vi "FlexMag - 23-03-2023.vi"() -> ()   [LabVIEW 2018] (continued)
        n1562 = local read "CH4_M3_D3_DO"() -> (w2043:bool)
        n1563 = feedback #54() -> (w2099:bool)  [unwired: 1 in]
        n1564 = Exclusive Or(1:w2102, 2:w2101) -> (0:w2098:bool)
        n1565 = feedback #55() -> (w2106:bool)  [unwired: 1 in]
        n1566 = Exclusive Or(1:w2103, 2:w2104) -> (0:w2107:bool)
        n1567 = feedback #56() -> (w2116:bool)  [unwired: 1 in]
        n1568 = Exclusive Or(1:w2113, 2:w2114) -> (0:w2117:bool)
        n1569 = feedback #57() -> (w2109:bool)  [unwired: 1 in]
        n1570 = Exclusive Or(1:w2112, 2:w2111) -> (0:w2108:bool)
        n1571 = feedback #58() -> (w2053:bool)  [unwired: 1 in]
        n1572 = Exclusive Or(1:w2056, 2:w2055) -> (0:w2052:bool)
        n1573 = feedback #59() -> (w2045:bool)  [unwired: 1 in]
        n1574 = Exclusive Or(1:w2042, 2:w2043) -> (0:w2046:bool)
        n1575 = feedback #60() -> (w2048:bool)  [unwired: 1 in]
        n1576 = Exclusive Or(1:w2051, 2:w2050) -> (0:w2047:bool)
        n1577 = case shown="True" w2098 {
          tunnel: w2099 -> [_ w2204]
          tunnel: [TRUE FALSE] -> w2100
          tunnel: [FALSE w2205] -> w2083
          frame False {
          }
          frame True {
            n1578 = call "Elapsed Time134"("Reset"=w2204) -> ("Elapsed Time (s)"=w2206:dbl)  [unwired: 11 in, 7 out]
            n1579 = Greater Or Equal?(x=w2206, y=5.0) -> (x >= y?=w2205:bool)
          }
        }
        n1580 = feedback-in #54(w2100) -> ()
        n1581 = case shown="True" w2107 {
          tunnel: w2106 -> [_ w2197]
          tunnel: [TRUE FALSE] -> w2105
          tunnel: [FALSE w2198] -> w2085
          frame False {
          }
          frame True {
            n1582 = call "Elapsed Time135"("Reset"=w2197) -> ("Elapsed Time (s)"=w2199:dbl)  [unwired: 11 in, 7 out]
            n1583 = Greater Or Equal?(x=w2199, y=5.0) -> (x >= y?=w2198:bool)
          }
        }
        n1584 = feedback-in #55(w2105) -> ()
        n1585 = case shown="True" w2117 {
          tunnel: w2116 -> [_ w2218]
          tunnel: [TRUE FALSE] -> w2115
          tunnel: [FALSE w2219] -> w2087
          frame False {
          }
          frame True {
            n1586 = call "Elapsed Time132"("Reset"=w2218) -> ("Elapsed Time (s)"=w2220:dbl)  [unwired: 11 in, 7 out]
            n1587 = Greater Or Equal?(x=w2220, y=5.0) -> (x >= y?=w2219:bool)
          }
        }
        n1588 = feedback-in #56(w2115) -> ()
        n1589 = case shown="True" w2108 {
          tunnel: w2109 -> [_ w2211]
          tunnel: [TRUE FALSE] -> w2110
          tunnel: [FALSE w2212] -> w2084
          frame False {
          }
          frame True {
            n1590 = call "Elapsed Time133"("Reset"=w2211) -> ("Elapsed Time (s)"=w2213:dbl)  [unwired: 11 in, 7 out]
            n1591 = Greater Or Equal?(x=w2213, y=5.0) -> (x >= y?=w2212:bool)
          }
        }
        n1592 = feedback-in #57(w2110) -> ()
        n1593 = case shown="True" w2052 {
          tunnel: w2053 -> [_ w2141]
          tunnel: [TRUE FALSE] -> w2054
          tunnel: [FALSE w2142] -> _
          frame False {
          }
          frame True {
            n1594 = call "Elapsed Time145"("Reset"=w2141) -> ("Elapsed Time (s)"=w2143:dbl)  [unwired: 11 in, 7 out]
            n1595 = Greater Or Equal?(x=w2143, y=5.0) -> (x >= y?=w2142:bool)
          }
        }
        n1596 = feedback-in #58(w2054) -> ()
        n1597 = case shown="True" w2046 {
          tunnel: w2045 -> [_ w2127]
          tunnel: [TRUE FALSE] -> w2044
          tunnel: [FALSE w2128] -> _
          frame False {
          }
          frame True {
            n1598 = call "Elapsed Time148"("Reset"=w2127) -> ("Elapsed Time (s)"=w2129:dbl)  [unwired: 11 in, 7 out]
            n1599 = Greater Or Equal?(x=w2129, y=5.0) -> (x >= y?=w2128:bool)
          }
        }
        n1600 = feedback-in #59(w2044) -> ()
        n1601 = case shown="True" w2047 {
          tunnel: w2048 -> [_ w2134]
          tunnel: [TRUE FALSE] -> w2049
          tunnel: [FALSE w2135] -> _
          frame False {
          }
          frame True {
            n1602 = call "Elapsed Time147"("Reset"=w2134) -> ("Elapsed Time (s)"=w2136:dbl)  [unwired: 11 in, 7 out]
            n1603 = Greater Or Equal?(x=w2136, y=5.0) -> (x >= y?=w2135:bool)
          }
        }
        n1604 = feedback-in #60(w2049) -> ()
        n1605 = local write "ch4_ch_vbv_fail"(w2085) -> ()
        n1606 = local write "ch4_mp_fail"(w2087) -> ()
        n1607 = local write "ch4_tp_bv_fail"(w2084) -> ()
        n1608 = local write "ch4_bg_bv_fail"(w2083) -> ()
        n1609 = local read "CH4_SRV1_Piston_Back_DO"() -> (w2075:bool)
        n1610 = local read "CH4_SRV1_Piston_Back_DI"() -> (w2076:bool)
        n1611 = local read "CH4_SRV1_Piston_For_DO"() -> (w2058:bool)
        n1612 = local read "CH4_SRV1_Piston_For_DI"() -> (w2057:bool)
        n1613 = local read "CH4_Trns_BP_Right_DO"() -> (w2039:bool)
        n1614 = local read "CH4_Trns_BP_Right_DI"() -> (w2040:bool)
        n1615 = local read "CH4_PetCool_Up_DO"() -> (w2068:bool)
        n1616 = local read "CH4_PetCool_Up_DI"() -> (w2067:bool)
        n1617 = local read "CH4_PetCool_Down_DO"() -> (w2065:bool)
        n1618 = local read "CH4_PetCool_Down_DI"() -> (w2066:bool)
        n1619 = local read "CH4_Cst_Fix_Down_DI"() -> (w2077:bool)
        n1620 = local read "CH4_PL_VBV_DO"() -> (w2091:bool)
        n1621 = local read "CH4_PL_VBV_DI"() -> (w2092:bool)
        n1622 = local read "CH4_SoV_Ar_DO"() -> (w2094:bool)
        n1623 = local read "CH4_SoV_Ar_DI"() -> (w2093:bool)
        n1624 = local read "CH4_Cst_Fix_DO"() -> (w2078:bool)
        n1625 = feedback #61() -> (w2089:bool)  [unwired: 1 in]
        n1626 = Exclusive Or(1:w2092, 2:w2091) -> (0:w2088:bool)
        n1627 = feedback #62() -> (w2096:bool)  [unwired: 1 in]
        n1628 = Exclusive Or(1:w2093, 2:w2094) -> (0:w2097:bool)
        n1629 = feedback #63() -> (w2080:bool)  [unwired: 1 in]
        n1630 = Exclusive Or(1:w2077, 2:w2078) -> (0:w2081:bool)
        n1631 = feedback #64() -> (w2073:bool)  [unwired: 1 in]
        n1632 = Exclusive Or(1:w2076, 2:w2075) -> (0:w2072:bool)
        n1633 = feedback #65() -> (w2060:bool)  [unwired: 1 in]
        n1634 = Exclusive Or(1:w2057, 2:w2058) -> (0:w2061:bool)
        n1635 = feedback #66() -> (w2063:bool)  [unwired: 1 in]
        n1636 = Exclusive Or(1:w2066, 2:w2065) -> (0:w2062:bool)
        n1637 = feedback #67() -> (w2070:bool)  [unwired: 1 in]
        n1638 = Exclusive Or(1:w2067, 2:w2068) -> (0:w2071:bool)
        n1639 = feedback #68() -> (w2037:bool)  [unwired: 1 in]
        n1640 = Exclusive Or(1:w2040, 2:w2039) -> (0:w2036:bool)
        n1641 = case shown="True" w2088 {
          tunnel: w2089 -> [_ w2190]
          tunnel: [TRUE FALSE] -> w2090
          tunnel: [FALSE w2191] -> w2086
          frame False {
          }
          frame True {
            n1642 = call "Elapsed Time136"("Reset"=w2190) -> ("Elapsed Time (s)"=w2192:dbl)  [unwired: 11 in, 7 out]
            n1643 = Greater Or Equal?(x=w2192, y=5.0) -> (x >= y?=w2191:bool)
          }
        }
        n1644 = feedback-in #61(w2090) -> ()
        n1645 = case shown="True" w2097 {
          tunnel: w2096 -> [_ w2183]
          tunnel: [TRUE FALSE] -> w2095
          tunnel: [FALSE w2184] -> w2082
          frame False {
          }
          frame True {
            n1646 = call "Elapsed Time137"("Reset"=w2183) -> ("Elapsed Time (s)"=w2185:dbl)  [unwired: 11 in, 7 out]
            n1647 = Greater Or Equal?(x=w2185, y=5.0) -> (x >= y?=w2184:bool)
          }
        }
        n1648 = feedback-in #62(w2095) -> ()
        n1649 = case shown="True" w2081 {
          tunnel: w2080 -> [_ w2176]
          tunnel: [TRUE FALSE] -> w2079
          tunnel: [FALSE w2177] -> _
          frame False {
          }
          frame True {
            n1650 = call "Elapsed Time140"("Reset"=w2176) -> ("Elapsed Time (s)"=w2178:dbl)  [unwired: 11 in, 7 out]
            n1651 = Greater Or Equal?(x=w2178, y=20.0) -> (x >= y?=w2177:bool)
          }
        }
        n1652 = feedback-in #63(w2079) -> ()
        n1653 = case shown="True" w2072 {
          tunnel: w2073 -> [_ w2169]
          tunnel: [TRUE FALSE] -> w2074
          tunnel: [FALSE w2170] -> _
          frame False {
          }
          frame True {
            n1654 = call "Elapsed Time141"("Reset"=w2169) -> ("Elapsed Time (s)"=w2171:dbl)  [unwired: 11 in, 7 out]
            n1655 = Greater Or Equal?(x=w2171, y=25.0) -> (x >= y?=w2170:bool)
          }
        }
        n1656 = feedback-in #64(w2074) -> ()
        n1657 = case shown="True" w2061 {
          tunnel: w2060 -> [_ w2148]
          tunnel: [TRUE FALSE] -> w2059
          tunnel: [FALSE w2149] -> _
          frame False {
          }
          frame True {
            n1658 = call "Elapsed Time144"("Reset"=w2148) -> ("Elapsed Time (s)"=w2150:dbl)  [unwired: 11 in, 7 out]
            n1659 = Greater Or Equal?(x=w2150, y=25.0) -> (x >= y?=w2149:bool)
          }
        }
        n1660 = feedback-in #65(w2059) -> ()
        n1661 = case shown="True" w2062 {
          tunnel: w2063 -> [_ w2162]
          tunnel: [TRUE FALSE] -> w2064
          tunnel: [FALSE w2163] -> _
          frame False {
          }
          frame True {
            n1662 = call "Elapsed Time142"("Reset"=w2162) -> ("Elapsed Time (s)"=w2164:dbl)  [unwired: 11 in, 7 out]
            n1663 = Greater Or Equal?(x=w2164, y=25.0) -> (x >= y?=w2163:bool)
          }
        }
        n1664 = feedback-in #66(w2064) -> ()
        n1665 = case shown="True" w2071 {
          tunnel: w2070 -> [_ w2155]
          tunnel: [TRUE FALSE] -> w2069
          tunnel: [FALSE w2156] -> _
          frame False {
          }
          frame True {
            n1666 = call "Elapsed Time143"("Reset"=w2155) -> ("Elapsed Time (s)"=w2157:dbl)  [unwired: 11 in, 7 out]
            n1667 = Greater Or Equal?(x=w2157, y=25.0) -> (x >= y?=w2156:bool)
          }
        }
        n1668 = feedback-in #67(w2069) -> ()
        n1669 = case shown="True" w2036 {
          tunnel: w2037 -> [_ w2120]
          tunnel: [TRUE FALSE] -> w2038
          tunnel: [FALSE w2121] -> w2041
          frame False {
          }
          frame True {
            n1670 = call "Elapsed Time149"("Reset"=w2120) -> ("Elapsed Time (s)"=w2122:dbl)  [unwired: 11 in, 7 out]
            n1671 = Greater Or Equal?(x=w2122, y=10.0) -> (x >= y?=w2121:bool)
          }
        }
        n1672 = feedback-in #68(w2038) -> ()
        n1673 = local write "ch4_gv_bp_right_fail"(w2041) -> ()
        n1674 = local write "ch4_pl_vbv_fail"(w2086) -> ()
        n1675 = local write "ch4_sov_fail"(w2082) -> ()
      }
    }
    n1676 = flat-sequence {
      frame #0 {
        n1677 = local read "CH3_Trns_Gv_Open_DI"() -> (w2328:bool)
        n1678 = local read "CH3_Trns_BP_Right_DI"() -> (w2329:bool)
        n1679 = local read "pcgv1 position"() -> (w2389:i32)
        n1680 = local read "CH1_Trns_Gv_Open_DI"() -> (w2367:bool)
        n1681 = local read "CH3_Trns_BP_Left_DI"() -> (w2330:bool)
        n1682 = local read "CH4_Trns_BP_Right_DI"() -> (w2264:bool)
        n1683 = local read "CH1_Trns_BP_Left_DI"() -> (w2351:bool)
        n1684 = local read "CH2_Trns_Gv_Open_DI"() -> (w2352:bool)
        n1685 = local read "Tp1_stop_cmnd"() -> (w2227:bool)
        n1686 = local read "CH2_Trns_BP_Right_DI"() -> (w2350:bool)
        n1687 = local read "Tp3_stop_cmnd"() -> (w2224:bool)
        n1688 = local read "pcgv3 position"() -> (w2324:i32)
        n1689 = local read "Tp2_stop_cmnd"() -> (w2223:bool)
        n1690 = local read "CH2_Trns_BP_Left_DI"() -> (w2349:bool)
        n1691 = local read "CH2_CH_ATM_DI"() -> (w2361:bool)
        n1692 = local read "CH1_CH_ATM_DI"() -> (w2394:bool)
        n1693 = local read "pcgv4 position"() -> (w2268:i32)
        n1694 = local read "pcgv2 position"() -> (w2356:i32)
        n1695 = local read "CH3_SoV_Ar_DI"() -> (w2327:bool)
        n1696 = local read "CH2_CH_VBV_DI"() -> (w2362:bool)
        n1697 = local read "CH2_PL_ATM_DI"() -> (w2360:bool)
        n1698 = local read "CH1_CH_VBV_DI"() -> (w2395:bool)
        n1699 = local read "CH1_PL_ATM_DI"() -> (w2392:bool)
        n1700 = local read "CH2_PL_VBV_DI"() -> (w2365:bool)
        n1701 = local read "CH1_PL_VBV_DI"() -> (w2393:bool)
        n1702 = local read "CH1_SoV_Ar_DI"() -> (w2368:bool)
        n1703 = local read "CH2_BG_BV_DI"() -> (w2363:bool)
        n1704 = local read "CH1_BG_BV_DI"() -> (w2396:bool)
        n1705 = local read "CH2_TP_BV_DI"() -> (w2364:bool)
        n1706 = local read "CH3_CH_ATM_DI"() -> (w2319:bool)
        n1707 = local read "CH4_SoV_Ar_DI"() -> (w2265:bool)
        n1708 = local read "CH1_TP_BV_DI"() -> (w2397:bool)
        n1709 = local read "CH3_CH_VBV_DI"() -> (w2318:bool)
        n1710 = local read "CH3_PL_ATM_DI"() -> (w2320:bool)
        n1711 = local read "CH2_SoV_Ar_DI"() -> (w2353:bool)
        n1712 = local read "CH3_PL_VBV_DI"() -> (w2315:bool)
        n1713 = local read "CH4_CH_ATM_DI"() -> (w2273:bool)
        n1714 = local read "CH3_BG_BV_DI"() -> (w2317:bool)
        n1715 = local read "CH2_MP_DI"() -> (w2366:bool)
        n1716 = local read "CH3_TP_BV_DI"() -> (w2316:bool)
        n1717 = local read "CH1_MP_DI"() -> (w2398:bool)
        n1718 = local read "CH2_CC_DI"() -> (w2359:bool)
        n1719 = local read "CH4_CH_VBV_DI"() -> (w2274:bool)
        n1720 = local read "CH4_PL_ATM_DI"() -> (w2272:bool)
        n1721 = local read "CH4_PL_VBV_DI"() -> (w2277:bool)
        n1722 = local read "CH4_BG_BV_DI"() -> (w2275:bool)
        n1723 = local read "CH4_TP_BV_DI"() -> (w2276:bool)
        n1724 = local read "CH3_MP_DI"() -> (w2314:bool)
        n1725 = local read "CH3_CC_DI"() -> (w2321:bool)
        n1726 = local read "CH4_MP_DI"() -> (w2278:bool)
        n1727 = local read "CH4_CC_DI"() -> (w2271:bool)
        n1728 = case shown="True" w2227 {
          tunnel: [w2417 w2420] -> w2228
          frame False {
            n1729 = local read "Tp1 speed gui"() -> (w2419:i32)
            n1730 = Greater?(x=w2419, y=250) -> (0:w2417:bool)
          }
          frame True {
            n1731 = local read "Tp1 speed gui"() -> (w2421:i32)
            n1732 = Greater?(x=w2421, y=400) -> (0:w2420:bool)
          }
        }
        n1733 = Greater?(x=w2389, y=10) -> (0:w2388:bool)
        n1734 = Greater?(x=w2389, y=90) -> (0:w2387:bool)
        n1735 = case shown="True" w2223 {
          tunnel: [w2399 w2402] -> w2229
          frame False {
            n1736 = local read "Tp2 speed gui"() -> (w2401:i32)
            n1737 = Greater?(x=w2401, y=250) -> (0:w2399:bool)
          }
          frame True {
            n1738 = local read "Tp2 speed gui"() -> (w2404:i32)
            n1739 = Greater?(x=w2404, y=400) -> (0:w2402:bool)
          }
        }
        n1740 = local write "ch3_sov_gui"(w2327) -> ()
        n1741 = local write "ch3_4_trns_gv_gui"(w2328) -> ()
        n1742 = local write "ch3_gv_bp_right_gui"(w2329) -> ()
        n1743 = local write "ch3_gv_bp_left_gui"(w2330) -> ()
        n1744 = Greater?(x=w2324, y=10) -> (0:w2323:bool)
        n1745 = Greater?(x=w2324, y=90) -> (0:w2322:bool)
        n1746 = local write "ch4_sov_gui"(w2265) -> ()
        n1747 = local write "ch4_gv_bp_right_gui"(w2264) -> ()
        n1748 = local write "ch2_mp_gui"(w2366) -> ()
        n1749 = local write "ch2_tp_bv_gui"(w2364) -> ()
        n1750 = local write "ch2_bg_bv_gui"(w2363) -> ()
        n1751 = local write "ch2_ch_vbv_gui"(w2362) -> ()
        n1752 = local write "ch2_ch_atm_gui"(w2361) -> ()
        n1753 = local write "ch2_pl_vbv_gui"(w2365) -> ()
        n1754 = local write "ch2_pl_atm_gui"(w2360) -> ()
        n1755 = local write "ch2_cc_gui"(w2359) -> ()
        n1756 = case shown="True" w2224 {
          tunnel: [w2405 w2408] -> w2230
          frame False {
            n1757 = local read "Tp3 speed gui"() -> (w2407:i32)
            n1758 = Greater?(x=w2407, y=250) -> (0:w2405:bool)
          }
          frame True {
            n1759 = local read "Tp3 speed gui"() -> (w2410:i32)
            n1760 = Greater?(x=w2410, y=400) -> (0:w2408:bool)
          }
        }
        n1761 = local write "ch1_sov_gui"(w2368) -> ()
        n1762 = local write "ch1_2_trns_gv_gui"(w2367) -> ()
        n1763 = local write "ch1_gv_bp_left_gui"(w2351) -> ()
        n1764 = local write "ch1_mp_gui"(w2398) -> ()
        n1765 = local write "ch1_tp_bv_gui"(w2397) -> ()
        n1766 = local write "ch1_bg_bv_gui"(w2396) -> ()
        n1767 = local write "ch1_ch_vbv_gui"(w2395) -> ()
        n1768 = local write "ch1_ch_atm_gui"(w2394) -> ()
        n1769 = local write "ch1_pl_vbv_gui"(w2393) -> ()
        n1770 = local write "ch1_pl_atm_gui"(w2392) -> ()
        n1771 = local write "ch2_sov_gui"(w2353) -> ()
        n1772 = local write "ch2_3_trns_gv_gui"(w2352) -> ()
        n1773 = local write "ch2_gv_bp_right_gui"(w2350) -> ()
        n1774 = local write "ch2_gv_bp_left_gui"(w2349) -> ()
        n1775 = Greater?(x=w2268, y=10) -> (0:w2269:bool)
        n1776 = Greater?(x=w2268, y=90) -> (0:w2270:bool)
        n1777 = Greater?(x=w2356, y=10) -> (0:w2357:bool)
        n1778 = Greater?(x=w2356, y=90) -> (0:w2358:bool)
        n1779 = local write "ch1_pcgv_half_gui"(w2388) -> ()
        n1780 = local write "ch1_pcgv_gui"(w2387) -> ()
        n1781 = local write "ch3_mp_gui"(w2314) -> ()
        n1782 = local write "ch3_tp_bv_gui"(w2316) -> ()
        n1783 = local write "ch3_bg_bv_gui"(w2317) -> ()
        n1784 = local write "ch3_ch_vbv_gui"(w2318) -> ()
        n1785 = local write "ch3_ch_atm_gui"(w2319) -> ()
        n1786 = local write "ch3_pl_vbv_gui"(w2315) -> ()
        n1787 = local write "ch3_pl_atm_gui"(w2320) -> ()
        n1788 = local write "ch3_cc_gui"(w2321) -> ()
        n1789 = local write "ch4_mp_gui"(w2278) -> ()
        n1790 = local write "ch4_tp_bv_gui"(w2276) -> ()
        n1791 = local write "ch4_bg_bv_gui"(w2275) -> ()
        n1792 = local write "ch4_ch_vbv_gui"(w2274) -> ()
        n1793 = local write "ch4_ch_atm_gui"(w2273) -> ()
        n1794 = local write "ch4_pl_vbv_gui"(w2277) -> ()
        n1795 = local write "ch4_pl_atm_gui"(w2272) -> ()
        n1796 = local write "ch4_cc_gui"(w2271) -> ()
        n1797 = local write "ch3_pcgv_half_gui"(w2323) -> ()
        n1798 = local write "ch3_pcgv_gui"(w2322) -> ()
        n1799 = local write "ch4_pcgv_half_gui"(w2269) -> ()
        n1800 = local write "ch4_pcgv_gui"(w2270) -> ()
        n1801 = local write "ch2_pcgv_half_gui"(w2357) -> ()
        n1802 = local write "ch2_pcgv_gui"(w2358) -> ()
        n1803 = local write "ch2_tp_gui"(w2229) -> ()
        n1804 = local write "ch1_tp_gui"(w2228) -> ()
        n1805 = local read "ch3 pl pg ai(V)"() -> (w2309:dbl)
        n1806 = local read "ch4 pl pg ai(V)"() -> (w2282:dbl)
        n1807 = local read "ch1 pl pg ai(V)"() -> (w2382:dbl)
        n1808 = local read "ch2 pl pg ai(V)"() -> (w2335:dbl)
        n1809 = local read "CH2_CC_DI"() -> (w2346:bool)
        n1810 = local write "ch3_tp_gui"(w2230) -> ()
        n1811 = local read "CH1_CC_DI"() -> (w2371:bool)
        n1812 = local read "CH3_CC_DI"() -> (w2298:bool)
        n1813 = local read "CH4_CC_DI"() -> (w2293:bool)
        n1814 = feedback #69() -> (w2311:bool)  [unwired: 1 in]
        n1815 = feedback #70() -> (w2280:bool)  [unwired: 1 in]
        n1816 = feedback #71() -> (w2347:bool)  [unwired: 1 in]
        n1817 = feedback #72() -> (w2370:bool)  [unwired: 1 in]
        n1818 = feedback #73() -> (w2384:bool)  [unwired: 1 in]
        n1819 = feedback #74() -> (w2333:bool)  [unwired: 1 in]
        n1820 = feedback #75() -> (w2297:bool)  [unwired: 1 in]
        n1821 = Less Or Equal?(x=w2309, y=0.5) -> (x <= y?=w2310:bool)
        n1822 = Less Or Equal?(x=w2282, y=0.5) -> (x <= y?=w2281:bool)
        n1823 = Less Or Equal?(x=w2382, y=0.5) -> (x <= y?=w2383:bool)
        n1824 = Less Or Equal?(x=w2335, y=0.5) -> (x <= y?=w2334:bool)
        n1825 = feedback #76() -> (w2294:bool)  [unwired: 1 in]
        n1826 = case shown="True" w2346 {
          tunnel: w2347 -> [_ w2534]
          tunnel: [TRUE w2533] -> w2348
          tunnel: [FALSE w2529] -> w2240
          tunnel: [FALSE w2528] -> w2331
          frame False {
          }
          frame True {
            n1827 = local read "ch2 cc ai(V)"() -> (w2531:dbl)
            n1828 = Less Or Equal?(x=w2531, y=0.5) -> (x <= y?=w2532:bool)
            n1829 = case shown="True" w2532 {
              tunnel: [TRUE FALSE] -> w2533
              tunnel: w2534 -> [_ w2538]
              tunnel: [FALSE w2539] -> w2529
              tunnel: [TRUE FALSE] -> w2528
              frame False {
              }
              frame True {
                n1830 = call "Elapsed Time69"("Reset"=w2538) -> ("Elapsed Time (s)"=w2541:dbl)  [unwired: 11 in, 7 out]
                n1831 = Greater Or Equal?(x=w2541, y=6.0) -> (x >= y?=w2539:bool)
              }
            }
          }
        }
        n1832 = feedback-in #71(w2348) -> ()
        n1833 = case shown="True" w2310 {
          tunnel: [TRUE FALSE] -> w2312
          tunnel: w2311 -> [_ w2519]
          tunnel: [FALSE w2520] -> w2306
          tunnel: [TRUE FALSE] -> w2307
          frame False {
          }
          frame True {
            n1834 = call "Elapsed Time71"("Reset"=w2519) -> ("Elapsed Time (s)"=w2522:dbl)  [unwired: 11 in, 7 out]
            n1835 = Greater Or Equal?(x=w2522, y=5.0) -> (x >= y?=w2520:bool)
          }
        }
        n1836 = feedback-in #69(w2312) -> ()
        n1837 = case shown="True" w2281 {
          tunnel: [TRUE FALSE] -> w2279
          tunnel: w2280 -> [_ w2482]
          tunnel: [FALSE w2483] -> w2285
          tunnel: [TRUE FALSE] -> w2284
          frame False {
          }
          frame True {
            n1838 = call "Elapsed Time74"("Reset"=w2482) -> ("Elapsed Time (s)"=w2485:dbl)  [unwired: 11 in, 7 out]
            n1839 = Greater Or Equal?(x=w2485, y=5.0) -> (x >= y?=w2483:bool)
          }
        }
        n1840 = feedback-in #70(w2279) -> ()
        n1841 = case shown="True" w2371 {
          tunnel: w2370 -> [_ w2571]
          tunnel: [TRUE w2570] -> w2369
          tunnel: [FALSE w2566] -> w2232
          tunnel: [FALSE w2565] -> w2386
          frame False {
          }
          frame True {
            n1842 = local read "ch1 cc ai(V)"() -> (w2568:dbl)
            n1843 = Less Or Equal?(x=w2568, y=0.5) -> (x <= y?=w2569:bool)
            n1844 = case shown="True" w2569 {
              tunnel: [TRUE FALSE] -> w2570
              tunnel: w2571 -> [_ w2575]
              tunnel: [FALSE w2576] -> w2566
              tunnel: [TRUE FALSE] -> w2565
              frame False {
              }
              frame True {
                n1845 = call "Elapsed Time45"("Reset"=w2575) -> ("Elapsed Time (s)"=w2578:dbl)  [unwired: 11 in, 7 out]
                n1846 = Greater Or Equal?(x=w2578, y=6.0) -> (x >= y?=w2576:bool)
              }
            }
          }
        }
        n1847 = feedback-in #72(w2369) -> ()
        n1848 = case shown="True" w2383 {
          tunnel: [TRUE FALSE] -> w2385
          tunnel: w2384 -> [_ w2593]
          tunnel: [FALSE w2594] -> w2379
          tunnel: [TRUE FALSE] -> w2380
          frame False {
          }
          frame True {
            n1849 = call "Elapsed Time46"("Reset"=w2593) -> ("Elapsed Time (s)"=w2596:dbl)  [unwired: 11 in, 7 out]
            n1850 = Greater Or Equal?(x=w2596, y=5.0) -> (x >= y?=w2594:bool)
          }
        }
        n1851 = feedback-in #73(w2385) -> ()
        n1852 = case shown="True" w2298 {
          tunnel: w2297 -> [_ w2497]
          tunnel: [TRUE w2496] -> w2296
          tunnel: [FALSE w2492] -> w2248
          tunnel: [FALSE w2491] -> w2313
          frame False {
          }
          frame True {
            n1853 = local read "ch3 cc ai(V)"() -> (w2494:dbl)
            n1854 = Less Or Equal?(x=w2494, y=0.5) -> (x <= y?=w2495:bool)
            n1855 = case shown="True" w2495 {
              tunnel: [TRUE FALSE] -> w2496
              tunnel: w2497 -> [_ w2501]
              tunnel: [FALSE w2502] -> w2492
              tunnel: [TRUE FALSE] -> w2491
              frame False {
              }
              frame True {
                n1856 = call "Elapsed Time73"("Reset"=w2501) -> ("Elapsed Time (s)"=w2504:dbl)  [unwired: 11 in, 7 out]
                n1857 = Greater Or Equal?(x=w2504, y=6.0) -> (x >= y?=w2502:bool)
              }
            }
          }
        }
        n1858 = feedback-in #75(w2296) -> ()
        n1859 = case shown="True" w2334 {
          tunnel: [TRUE FALSE] -> w2332
          tunnel: w2333 -> [_ w2556]
          tunnel: [FALSE w2557] -> w2338
          tunnel: [TRUE FALSE] -> w2337
          frame False {
          }
          frame True {
            n1860 = call "Elapsed Time67"("Reset"=w2556) -> ("Elapsed Time (s)"=w2559:dbl)  [unwired: 11 in, 7 out]
            n1861 = Greater Or Equal?(x=w2559, y=5.0) -> (x >= y?=w2557:bool)
          }
        }
        n1862 = feedback-in #74(w2332) -> ()
        n1863 = local read "CH2_CC_DO"() -> (w2243:bool)
        n1864 = local read "CH2_CC_DI"() -> (w2244:bool)
        n1865 = local read "CH1_CC_DO"() -> (w2235:bool)
        n1866 = local read "CH1_CC_DI"() -> (w2236:bool)
        n1867 = local read "CH3_CC_DO"() -> (w2253:bool)
        n1868 = local read "CH3_CC_DI"() -> (w2252:bool)
        n1869 = local read "Tp4_stop_cmnd"() -> (w2226:bool)
        n1870 = case shown="True" w2293 {
          tunnel: w2294 -> [_ w2460]
          tunnel: [TRUE w2459] -> w2295
          tunnel: [FALSE w2455] -> w2257
          tunnel: [FALSE w2454] -> w2258
          frame False {
          }
          frame True {
            n1871 = local read "ch4 cc ai(V)"() -> (w2457:dbl)
            n1872 = Less Or Equal?(x=w2457, y=0.5) -> (x <= y?=w2458:bool)
            n1873 = case shown="True" w2458 {
              tunnel: [TRUE FALSE] -> w2459
              tunnel: w2460 -> [_ w2464]
              tunnel: [FALSE w2465] -> w2455
              tunnel: [TRUE FALSE] -> w2454
              frame False {
              }
              frame True {
                n1874 = call "Elapsed Time76"("Reset"=w2464) -> ("Elapsed Time (s)"=w2467:dbl)  [unwired: 11 in, 7 out]
                n1875 = Greater Or Equal?(x=w2467, y=6.0) -> (x >= y?=w2465:bool)
              }
            }
          }
        }
        n1876 = feedback-in #76(w2295) -> ()
        n1877 = local read "CH4_CC_DO"() -> (w2260:bool)
        n1878 = local read "CH4_CC_DI"() -> (w2261:bool)
        n1879 = feedback #77() -> (w2246:bool)  [unwired: 1 in]
        n1880 = Exclusive Or(1:w2244, 2:w2243) -> (0:w2245:bool)
        n1881 = feedback #78() -> (w2238:bool)  [unwired: 1 in]
        n1882 = Exclusive Or(1:w2236, 2:w2235) -> (0:w2237:bool)
        n1883 = feedback #79() -> (w2250:bool)  [unwired: 1 in]
        n1884 = Exclusive Or(1:w2252, 2:w2253) -> (0:w2251:bool)
        n1885 = case shown="True" w2226 {
          tunnel: [w2411 w2414] -> w2225
          frame False {
            n1886 = local read "Tp4 speed gui"() -> (w2413:i32)
            n1887 = Greater?(x=w2413, y=250) -> (0:w2411:bool)
          }
          frame True {
            n1888 = local read "Tp4 speed gui"() -> (w2416:i32)
            n1889 = Greater?(x=w2416, y=400) -> (0:w2414:bool)
          }
        }
        n1890 = feedback #80() -> (w2263:bool)  [unwired: 1 in]
        n1891 = Exclusive Or(1:w2261, 2:w2260) -> (0:w2262:bool)
        n1892 = case shown="True" w2245 {
          tunnel: w2246 -> [_ w2432]
          tunnel: [TRUE FALSE] -> w2242
          tunnel: [FALSE w2433] -> w2241
          frame False {
          }
          frame True {
            n1893 = call "Elapsed Time86"("Reset"=w2432) -> ("Elapsed Time (s)"=w2434:dbl)  [unwired: 11 in, 7 out]
            n1894 = Greater Or Equal?(x=w2434, y=5.0) -> (x >= y?=w2433:bool)
          }
        }
        n1895 = feedback-in #77(w2242) -> ()
        n1896 = case shown="True" w2237 {
          tunnel: w2238 -> [_ w2425]
          tunnel: [TRUE FALSE] -> w2234
          tunnel: [FALSE w2426] -> w2233
          frame False {
          }
          frame True {
            n1897 = call "Elapsed Time87"("Reset"=w2425) -> ("Elapsed Time (s)"=w2427:dbl)  [unwired: 11 in, 7 out]
            n1898 = Greater Or Equal?(x=w2427, y=5.0) -> (x >= y?=w2426:bool)
          }
        }
        n1899 = feedback-in #78(w2234) -> ()
        n1900 = case shown="True" w2251 {
          tunnel: w2250 -> [_ w2439]
          tunnel: [TRUE FALSE] -> w2254
          tunnel: [FALSE w2440] -> w2249
          frame False {
          }
          frame True {
            n1901 = call "Elapsed Time85"("Reset"=w2439) -> ("Elapsed Time (s)"=w2441:dbl)  [unwired: 11 in, 7 out]
            n1902 = Greater Or Equal?(x=w2441, y=5.0) -> (x >= y?=w2440:bool)
          }
        }
        n1903 = feedback-in #79(w2254) -> ()
        n1904 = local write "ch3_pl_pg_fail"(w2306) -> ()
        n1905 = local write "ch3_pl_pg_gui"(w2307) -> ()
        n1906 = local write "ch4_pl_pg_fail"(w2285) -> ()
        n1907 = local write "ch4_pl_pg_gui"(w2284) -> ()
        n1908 = local write "ch1_pl_pg_fail"(w2379) -> ()
        n1909 = local write "ch1_pl_pg_gui"(w2380) -> ()
        n1910 = local write "ch2_pl_pg_fail"(w2338) -> ()
        n1911 = local write "ch2_pl_pg_gui"(w2337) -> ()
        n1912 = case shown="True" w2262 {
          tunnel: w2263 -> [_ w2446]
          tunnel: [TRUE FALSE] -> w2259
          tunnel: [FALSE w2447] -> w2256
          frame False {
          }
          frame True {
            n1913 = call "Elapsed Time66"("Reset"=w2446) -> ("Elapsed Time (s)"=w2448:dbl)  [unwired: 11 in, 7 out]
            n1914 = Greater Or Equal?(x=w2448, y=5.0) -> (x >= y?=w2447:bool)
          }
        }
        n1915 = feedback-in #80(w2259) -> ()
        n1916 = local read "ch3 ch pg ai(V)"() -> (w2302:dbl)
        n1917 = local read "ch4 ch pg ai(V)"() -> (w2289:dbl)
        n1918 = local read "ch2 ch pg ai(V)"() -> (w2342:dbl)
        n1919 = local read "ch1 ch pg ai(V)"() -> (w2375:dbl)
        n1920 = local write "ch4_tp_gui"(w2225) -> ()
        n1921 = local write "ch1_cc_gui"(w2386) -> ()
        n1922 = local write "ch2_cc_gui"(w2331) -> ()
        n1923 = local write "ch3_cc_gui"(w2313) -> ()
        n1924 = feedback #81() -> (w2300:bool)  [unwired: 1 in]
        n1925 = feedback #82() -> (w2291:bool)  [unwired: 1 in]
        n1926 = feedback #83() -> (w2344:bool)  [unwired: 1 in]
        n1927 = feedback #84() -> (w2373:bool)  [unwired: 1 in]
        n1928 = Less Or Equal?(x=w2302, y=0.5) -> (x <= y?=w2301:bool)
        n1929 = Less Or Equal?(x=w2289, y=0.5) -> (x <= y?=w2290:bool)
        n1930 = Less Or Equal?(x=w2342, y=0.5) -> (x <= y?=w2343:bool)
        n1931 = Less Or Equal?(x=w2375, y=0.5) -> (x <= y?=w2374:bool)
        n1932 = local write "ch4_cc_gui"(w2258) -> ()
        n1933 = case shown="True" w2301 {
          tunnel: [TRUE FALSE] -> w2299
          tunnel: w2300 -> [_ w2510]
          tunnel: [FALSE w2511] -> w2305
          tunnel: [TRUE FALSE] -> w2304
          frame False {
          }
          frame True {
            n1934 = call "Elapsed Time72"("Reset"=w2510) -> ("Elapsed Time (s)"=w2513:dbl)  [unwired: 11 in, 7 out]
            n1935 = Greater Or Equal?(x=w2513, y=5.0) -> (x >= y?=w2511:bool)
          }
        }
        n1936 = feedback-in #81(w2299) -> ()
        n1937 = case shown="True" w2290 {
          tunnel: [TRUE FALSE] -> w2292
          tunnel: w2291 -> [_ w2473]
          tunnel: [FALSE w2474] -> w2286
          tunnel: [TRUE FALSE] -> w2287
          frame False {
          }
          frame True {
            n1938 = call "Elapsed Time75"("Reset"=w2473) -> ("Elapsed Time (s)"=w2476:dbl)  [unwired: 11 in, 7 out]
            n1939 = Greater Or Equal?(x=w2476, y=5.0) -> (x >= y?=w2474:bool)
          }
        }
        n1940 = feedback-in #82(w2292) -> ()
        n1941 = case shown="True" w2343 {
          tunnel: [TRUE FALSE] -> w2345
          tunnel: w2344 -> [_ w2547]
          tunnel: [FALSE w2548] -> w2339
          tunnel: [TRUE FALSE] -> w2340
          frame False {
          }
          frame True {
            n1942 = call "Elapsed Time68"("Reset"=w2547) -> ("Elapsed Time (s)"=w2550:dbl)  [unwired: 11 in, 7 out]
            n1943 = Greater Or Equal?(x=w2550, y=5.0) -> (x >= y?=w2548:bool)
          }
        }
        n1944 = feedback-in #83(w2345) -> ()
        n1945 = case shown="True" w2374 {
          tunnel: [TRUE FALSE] -> w2372
          tunnel: w2373 -> [_ w2584]
          tunnel: [FALSE w2585] -> w2378
          tunnel: [TRUE FALSE] -> w2377
          frame False {
          }
          frame True {
            n1946 = call "Elapsed Time47"("Reset"=w2584) -> ("Elapsed Time (s)"=w2587:dbl)  [unwired: 11 in, 7 out]
            n1947 = Greater Or Equal?(x=w2587, y=5.0) -> (x >= y?=w2585:bool)
          }
        }
        n1948 = feedback-in #84(w2372) -> ()
        n1949 = Or(x=w2232, y=w2233) -> (x .or. y?=w2231:bool)
        n1950 = Or(x=w2240, y=w2241) -> (x .or. y?=w2239:bool)
        n1951 = Or(x=w2248, y=w2249) -> (x .or. y?=w2247:bool)
        n1952 = local write "ch1_cc_fail"(w2231) -> ()
        n1953 = local write "ch2_cc_fail"(w2239) -> ()
        n1954 = Or(x=w2257, y=w2256) -> (x .or. y?=w2255:bool)
        n1955 = local write "ch3_cc_fail"(w2247) -> ()
        n1956 = local write "ch4_cc_fail"(w2255) -> ()
        n1957 = local write "ch3_ch_pg_gui"(w2304) -> ()
        n1958 = local write "ch3_ch_pg_fail"(w2305) -> ()
        n1959 = local write "ch4_ch_pg_gui"(w2287) -> ()
        n1960 = local write "ch4_ch_pg_fail"(w2286) -> ()
        n1961 = local write "ch2_ch_pg_gui"(w2340) -> ()
        n1962 = local write "ch2_ch_pg_fail"(w2339) -> ()
        n1963 = local write "ch1_ch_pg_gui"(w2377) -> ()
        n1964 = local write "ch1_ch_pg_fail"(w2378) -> ()
      }
    }
    n1965 = Wait Until Next ms Multiple(millisecond multiple=u32 300) -> ()  [unwired: 1 out]
  }
  n1966 = local write "Tp4_stop_cmnd"(w19) -> ()
  n1967 = local write "Tp3_stop_cmnd"(w19) -> ()
  n1968 = local write "Tp2_stop_cmnd"(w19) -> ()
  n1969 = local write "Tp1_stop_cmnd"(w19) -> ()
  n1970 = while {
    stop <- FALSE stop-if-true
    n1971 = stacked-sequence {
      seq-local: [w2602 _ _ _ _ _ _] -> [_ w3296 _ _ _ _ _]
      seq-local: [_ _ _ _ w4002 _ _] -> [_ _ _ _ _ _ w5167]
      seq-local: [_ w3019 _ _ _ _ _] -> [_ _ _ _ _ _ w5165]
      seq-local: [_ _ _ _ w3970 _ _] -> [_ _ _ _ _ _ w5158]
      frame #0 {
        n1972 = local read "tp vbv on jpeg"() -> (w2609:u32[][])
        n1973 = local read "pl atm on jpeg"() -> (w2615:u32[][])
        n1974 = local read "pl atm fail jpeg"() -> (w2614:u32[][])
        n1975 = local read "pl pg on jpeg"() -> (w2613:u32[][])
        n1976 = local read "tp vbv fail jpeg"() -> (w2608:u32[][])
        n1977 = local read "pl pg fail jpeg"() -> (w2612:u32[][])
        n1978 = local read "pc gv half jpeg"() -> (w2603:u32[][])
        n1979 = local read "pc gv on jpeg"() -> (w2604:u32[][])
        n1980 = local read "pc gv fail jpeg"() -> (w2605:u32[][])
        n1981 = local read "tp start jpeg"() -> (w2607:u32[][])
        n1982 = local read "main screen jpeg"() -> (w2620:u32[][])
        n1983 = local read "mp on jpeg"() -> (w2619:u32[][])
        n1984 = local read "mp fail jpeg"() -> (w2618:u32[][])
        n1985 = local read "tp fail jpeg"() -> (w2606:u32[][])
        n1986 = local read "tp bv fail jpeg"() -> (w2610:u32[][])
        n1987 = local read "pl vbv on jpeg"() -> (w2617:u32[][])
        n1988 = local read "pl vbv fail jpeg"() -> (w2616:u32[][])
        n1989 = local read "tp bv on jpeg"() -> (w2611:u32[][])
        n1990 = Build Array(FALSE, "ch2_mp_gui", "ch2_mp_fail") -> (w2902:bool[])
        n1991 = Build Array(FALSE, "ch3_mp_gui", "ch3_mp_fail") -> (w2891:bool[])
        n1992 = Build Array(FALSE, "ch4_mp_gui", "ch4_mp_fail") -> (w2885:bool[])
        n1993 = Build Array(FALSE, "ch1_pl_vbv_gui", "ch1_pl_vbv_fail") -> (w2872:bool[])
        n1994 = Build Array(FALSE, "ch1_pl_atm_gui", "ch1_pl_atm_fail") -> (w2808:bool[])
        n1995 = Build Array(FALSE, "ch1_pl_pg_gui", "ch1_pl_pg_fail") -> (w2800:bool[])
        n1996 = Build Array(FALSE, "ch3_pl_vbv_gui", "ch3_pl_vbv_fail") -> (w2861:bool[])
        n1997 = Build Array(FALSE, "ch1_tp_gui", "ch1_tp_fail") -> (w2668:bool[])
        n1998 = Build Array(FALSE, "ch1_tp_bv_gui", "ch1_tp_bv_fail") -> (w2740:bool[])
        n1999 = Build Array(FALSE, "ch1_ch_vbv_gui", "ch1_ch_vbv_fail") -> (w2726:bool[])
        n2000 = Build Array(FALSE, "ch4_pl_vbv_gui", "ch4_pl_vbv_fail") -> (w2857:bool[])
        n2001 = Build Array(FALSE, "ch3_pl_atm_gui", "ch3_pl_atm_fail") -> (w2819:bool[])
        n2002 = Build Array(FALSE, "ch3_pl_pg_gui", "ch3_pl_pg_fail") -> (w2789:bool[])
        n2003 = Build Array(FALSE, "ch3_tp_gui", "ch3_tp_fail") -> (w2679:bool[])
        n2004 = Build Array(FALSE, "ch3_tp_bv_gui", "ch3_tp_bv_fail") -> (w2751:bool[])
        n2005 = Build Array(FALSE, "ch3_ch_vbv_gui", "ch3_ch_vbv_fail") -> (w2715:bool[])
        n2006 = Build Array(FALSE, "ch2_pl_vbv_gui", "ch2_pl_vbv_fail") -> (w2868:bool[])
        n2007 = Build Array(FALSE, "ch4_pl_atm_gui", "ch4_pl_atm_fail") -> (w2823:bool[])
        n2008 = Build Array(FALSE, "ch4_pl_pg_gui", "ch4_pl_pg_fail") -> (w2785:bool[])
        n2009 = Build Array(FALSE, "ch1_mp_gui", "ch1_mp_fail") -> (w2910:bool[])
        n2010 = Build Array(FALSE, "ch4_tp_gui", "ch4_tp_fail") -> (w2683:bool[])
        n2011 = Build Array(FALSE, "ch4_tp_bv_gui", "ch4_tp_bv_fail") -> (w2755:bool[])
        n2012 = Build Array(FALSE, "ch4_ch_vbv_gui", "ch4_ch_vbv_fail") -> (w2711:bool[])
        n2013 = Build Array(FALSE, "ch2_pl_atm_gui", "ch2_pl_atm_fail") -> (w2812:bool[])
        n2014 = Build Array(FALSE, "ch2_pl_pg_gui", "ch2_pl_pg_fail") -> (w2796:bool[])
        n2015 = Build Array(FALSE, "ch2_tp_gui", "ch2_tp_fail") -> (w2672:bool[])
        n2016 = Build Array(FALSE, "ch2_tp_bv_gui", "ch2_tp_bv_fail") -> (w2744:bool[])
        n2017 = Build Array(FALSE, "ch2_ch_vbv_gui", "ch2_ch_vbv_fail") -> (w2722:bool[])
        n2018 = Boolean Array To Number(Boolean array=w2902) -> (number=w2901:u32)
        n2019 = Boolean Array To Number(Boolean array=w2891) -> (number=w2892:u32)
        n2020 = Boolean Array To Number(Boolean array=w2885) -> (number=w2884:u32)
        n2021 = Build Array(FALSE, "ch1_pcgv_half_gui", "ch1_pcgv_gui", "ch1_pcgv_fail") -> (w2653:bool[])
        n2022 = Build Array(FALSE, "ch3_pcgv_half_gui", "ch3_pcgv_gui", "ch3_pcgv_fail") -> (w2642:bool[])
        n2023 = Build Array(FALSE, "ch2_pcgv_half_gui", "ch2_pcgv_gui", "ch2_pcgv_fail") -> (w2649:bool[])
        n2024 = Boolean Array To Number(Boolean array=w2872) -> (number=w2871:u32)
        n2025 = Boolean Array To Number(Boolean array=w2808) -> (number=w2809:u32)
        n2026 = Boolean Array To Number(Boolean array=w2800) -> (number=w2799:u32)
        n2027 = Build Array(FALSE, "ch4_pcgv_half_gui", "ch4_pcgv_gui", "ch4_pcgv_fail") -> (w2638:bool[])
        n2028 = Boolean Array To Number(Boolean array=w2861) -> (number=w2860:u32)
        n2029 = Boolean Array To Number(Boolean array=w2668) -> (number=w2669:u32)
        n2030 = Boolean Array To Number(Boolean array=w2740) -> (number=w2741:u32)
        n2031 = Boolean Array To Number(Boolean array=w2726) -> (number=w2725:u32)
        n2032 = Boolean Array To Number(Boolean array=w2857) -> (number=w2858:u32)
        n2033 = Boolean Array To Number(Boolean array=w2819) -> (number=w2820:u32)
        n2034 = Boolean Array To Number(Boolean array=w2789) -> (number=w2788:u32)
        n2035 = Boolean Array To Number(Boolean array=w2679) -> (number=w2680:u32)
        n2036 = Boolean Array To Number(Boolean array=w2751) -> (number=w2752:u32)
        n2037 = Boolean Array To Number(Boolean array=w2715) -> (number=w2714:u32)
        n2038 = Boolean Array To Number(Boolean array=w2868) -> (number=w2869:u32)
        n2039 = Boolean Array To Number(Boolean array=w2823) -> (number=w2822:u32)
        n2040 = Boolean Array To Number(Boolean array=w2785) -> (number=w2786:u32)
        n2041 = Boolean Array To Number(Boolean array=w2910) -> (number=w2911:u32)
        n2042 = Boolean Array To Number(Boolean array=w2683) -> (number=w2682:u32)
        n2043 = Boolean Array To Number(Boolean array=w2755) -> (number=w2754:u32)
        n2044 = Boolean Array To Number(Boolean array=w2711) -> (number=w2712:u32)
        n2045 = Boolean Array To Number(Boolean array=w2812) -> (number=w2811:u32)
        n2046 = Boolean Array To Number(Boolean array=w2796) -> (number=w2797:u32)
        n2047 = Boolean Array To Number(Boolean array=w2672) -> (number=w2671:u32)
        n2048 = Boolean Array To Number(Boolean array=w2744) -> (number=w2743:u32)
        n2049 = Boolean Array To Number(Boolean array=w2722) -> (number=w2723:u32)
        n2050 = Mantissa & Exponent(0:w2901) -> (2:w2897:dbl)  [unwired: 1 out]
        n2051 = Mantissa & Exponent(0:w2892) -> (2:w2886:dbl)  [unwired: 1 out]
        n2052 = Mantissa & Exponent(0:w2884) -> (2:w2880:dbl)  [unwired: 1 out]
        n2053 = Boolean Array To Number(Boolean array=w2653) -> (number=w2652:u32)
        n2054 = Boolean Array To Number(Boolean array=w2642) -> (number=w2641:u32)
        n2055 = Boolean Array To Number(Boolean array=w2649) -> (number=w2650:u32)
        n2056 = Mantissa & Exponent(0:w2871) -> (2:w2870:dbl)  [unwired: 1 out]
        n2057 = Mantissa & Exponent(0:w2809) -> (2:w2810:dbl)  [unwired: 1 out]
        n2058 = Mantissa & Exponent(0:w2799) -> (2:w2798:dbl)  [unwired: 1 out]
        n2059 = Mantissa & Exponent(0:w2860) -> (2:w2859:dbl)  [unwired: 1 out]
        n2060 = Mantissa & Exponent(0:w2669) -> (2:w2670:dbl)  [unwired: 1 out]
        n2061 = Mantissa & Exponent(0:w2741) -> (2:w2742:dbl)  [unwired: 1 out]
        n2062 = Mantissa & Exponent(0:w2725) -> (2:w2724:dbl)  [unwired: 1 out]
        n2063 = Mantissa & Exponent(0:w2858) -> (2:w2854:dbl)  [unwired: 1 out]
        n2064 = Mantissa & Exponent(0:w2820) -> (2:w2821:dbl)  [unwired: 1 out]
        n2065 = Mantissa & Exponent(0:w2788) -> (2:w2787:dbl)  [unwired: 1 out]
        n2066 = Mantissa & Exponent(0:w2680) -> (2:w2681:dbl)  [unwired: 1 out]
        n2067 = Mantissa & Exponent(0:w2752) -> (2:w2753:dbl)  [unwired: 1 out]
        n2068 = Mantissa & Exponent(0:w2714) -> (2:w2713:dbl)  [unwired: 1 out]
        n2069 = Mantissa & Exponent(0:w2869) -> (2:w2864:dbl)  [unwired: 1 out]
        n2070 = Mantissa & Exponent(0:w2822) -> (2:w2826:dbl)  [unwired: 1 out]
        n2071 = Mantissa & Exponent(0:w2786) -> (2:w2782:dbl)  [unwired: 1 out]
        n2072 = Mantissa & Exponent(0:w2911) -> (2:w2906:dbl)  [unwired: 1 out]
        n2073 = Mantissa & Exponent(0:w2682) -> (2:w2686:dbl)  [unwired: 1 out]
        n2074 = Mantissa & Exponent(0:w2754) -> (2:w2758:dbl)  [unwired: 1 out]
        n2075 = Mantissa & Exponent(0:w2712) -> (2:w2708:dbl)  [unwired: 1 out]
        n2076 = Boolean Array To Number(Boolean array=w2638) -> (number=w2639:u32)
        n2077 = Mantissa & Exponent(0:w2811) -> (2:w2816:dbl)  [unwired: 1 out]
        n2078 = Mantissa & Exponent(0:w2797) -> (2:w2792:dbl)  [unwired: 1 out]
        n2079 = Mantissa & Exponent(0:w2671) -> (2:w2676:dbl)  [unwired: 1 out]
        n2080 = Mantissa & Exponent(0:w2743) -> (2:w2748:dbl)  [unwired: 1 out]
        n2081 = Mantissa & Exponent(0:w2723) -> (2:w2718:dbl)  [unwired: 1 out]
        n2082 = Mantissa & Exponent(0:w2652) -> (2:w2651:dbl)  [unwired: 1 out]
        n2083 = Mantissa & Exponent(0:w2641) -> (2:w2640:dbl)  [unwired: 1 out]
        n2084 = Mantissa & Exponent(0:w2650) -> (2:w2645:dbl)  [unwired: 1 out]
        n2085 = Mantissa & Exponent(0:w2639) -> (2:w2635:dbl)  [unwired: 1 out]
        n2086 = case shown="0, Default" w2906 {
          tunnel: w2619 -> [_ w3010 _]
          tunnel: w2618 -> [_ _ w3011]
          tunnel: [u32[][] [] ("24-bit pixmap") w3010 w3011] -> w2904
          frame 0, Default {
          }
          frame 1 {
          }
          frame 2 {
          }
        }
        n2087 = case shown="2" w2886 {
          tunnel: w2619 -> [_ w3004 _]
          tunnel: w2618 -> [_ _ w3005]
          tunnel: [u32[][] [] ("24-bit pixmap") w3004 w3005] -> w2879
          frame 0, Default {
          }
          frame 1 {
          }
          frame 2 {
          }
        }
        n2088 = case shown="2" w2897 {
          tunnel: w2619 -> [_ w3007 _]
          tunnel: w2618 -> [_ _ w3008]
          tunnel: [u32[][] [] ("24-bit pixmap") w3007 w3008] -> w2895
          frame 0, Default {
          }
          frame 1 {
          }
          frame 2 {
          }
        }
        n2089 = case shown="0, Default" w2880 {
          tunnel: w2619 -> [_ w3001 _]
          tunnel: w2618 -> [_ _ w3002]
          tunnel: [u32[][] [] ("24-bit pixmap") w3001 w3002] -> w2877
          frame 0, Default {
          }
          frame 1 {
          }
          frame 2 {
          }
        }
        n2090 = case shown="0, Default" w2864 {
          tunnel: w2617 -> [_ w2995 _]
          tunnel: w2616 -> [_ _ w2996]
          tunnel: [u32[][] [] ("24-bit pixmap") w2995 w2996] -> w2847
          frame 0, Default {
          }
          frame 1 {
          }
          frame 2 {
          }
        }
        n2091 = case shown="0, Default" w2854 {
          tunnel: w2617 -> [_ w2989 _]
          tunnel: w2616 -> [_ _ w2990]
          tunnel: [u32[][] [] ("24-bit pixmap") w2989 w2990] -> w2843
          frame 0, Default {
          }
          frame 1 {
          }
          frame 2 {
          }
        }
        n2092 = case shown="0, Default" w2870 {
          tunnel: w2617 -> [_ w2998 _]
          tunnel: w2616 -> [_ _ w2999]
          tunnel: [u32[][] [] ("24-bit pixmap") w2998 w2999] -> w2848
          frame 0, Default {
          }
          frame 1 {
          }
          frame 2 {
          }
        }
        n2093 = case shown="0, Default" w2859 {
          tunnel: w2617 -> [_ w2992 _]
          tunnel: w2616 -> [_ _ w2993]
          tunnel: [u32[][] [] ("24-bit pixmap") w2992 w2993] -> w2844
          frame 0, Default {
          }
          frame 1 {
          }
          frame 2 {
          }
        }
        n2094 = case shown="0, Default" w2816 {
          tunnel: w2615 -> [_ w2983 _]
          tunnel: w2614 -> [_ _ w2984]
          tunnel: [u32[][] [] ("24-bit pixmap") w2983 w2984] -> w2832
          frame 0, Default {
          }
          frame 1 {
          }
          frame 2 {
          }
        }
        n2095 = case shown="0, Default" w2826 {
          tunnel: w2615 -> [_ w2977 _]
          tunnel: w2614 -> [_ _ w2978]
          tunnel: [u32[][] [] ("24-bit pixmap") w2977 w2978] -> w2836
          frame 0, Default {
          }
          frame 1 {
          }
          frame 2 {
          }
        }
        n2096 = case shown="0, Default" w2792 {
          tunnel: w2613 -> [_ w2971 _]
          tunnel: w2612 -> [_ _ w2972]
          tunnel: [u32[][] [] ("24-bit pixmap") w2971 w2972] -> w2776
          frame 0, Default {
          }
          frame 1 {
          }
          frame 2 {
          }
        }
        n2097 = case shown="0, Default" w2782 {
          tunnel: w2613 -> [_ w2965 _]
          tunnel: w2612 -> [_ _ w2966]
          tunnel: [u32[][] [] ("24-bit pixmap") w2965 w2966] -> w2772
          frame 0, Default {
          }
          frame 1 {
          }
          frame 2 {
          }
        }
        n2098 = case shown="3" w2645 {
          tunnel: w2603 -> [_ w2921 _ _]
          tunnel: w2604 -> [_ _ w2922 _]
          tunnel: [u32[][] [] ("24-bit pixmap") w2921 w2922 w2923] -> w2630
          tunnel: w2605 -> [_ _ _ w2923]
          frame 0, Default {
          }
          frame 1 {
          }
          frame 2 {
          }
          frame 3 {
          }
        }
        n2099 = case shown="0, Default" w2810 {
          tunnel: w2615 -> [_ w2986 _]
          tunnel: w2614 -> [_ _ w2987]
          tunnel: [u32[][] [] ("24-bit pixmap") w2986 w2987] -> w2831
          frame 0, Default {
          }
          frame 1 {
          }
          frame 2 {
          }
        }
        n2100 = case shown="0, Default" w2821 {
          tunnel: w2615 -> [_ w2980 _]
          tunnel: w2614 -> [_ _ w2981]
          tunnel: [u32[][] [] ("24-bit pixmap") w2980 w2981] -> w2835
          frame 0, Default {
          }
          frame 1 {
          }
          frame 2 {
          }
        }
        n2101 = case shown="0, Default" w2798 {
          tunnel: w2613 -> [_ w2974 _]
          tunnel: w2612 -> [_ _ w2975]
          tunnel: [u32[][] [] ("24-bit pixmap") w2974 w2975] -> w2777
          frame 0, Default {
          }
          frame 1 {
          }
          frame 2 {
          }
        }
        n2102 = case shown="0, Default" w2787 {
          tunnel: w2613 -> [_ w2968 _]
          tunnel: w2612 -> [_ _ w2969]
          tunnel: [u32[][] [] ("24-bit pixmap") w2968 w2969] -> w2773
          frame 0, Default {
          }
          frame 1 {
          }
          frame 2 {
          }
        }
        n2103 = case shown="0, Default" w2676 {
          tunnel: w2607 -> [_ w2935 _]
          tunnel: w2606 -> [_ _ w2936]
          tunnel: [u32[][] [] ("24-bit pixmap") w2935 w2936] -> w2692
          frame 0, Default {
          }
          frame 1 {
          }
          frame 2 {
          }
        }
        n2104 = case shown="0, Default" w2686 {
          tunnel: w2607 -> [_ w2929 _]
          tunnel: w2606 -> [_ _ w2930]
          tunnel: [u32[][] [] ("24-bit pixmap") w2929 w2930] -> w2694
          frame 0, Default {
          }
          frame 1 {
          }
          frame 2 {
          }
        }
        n2105 = case shown="3" w2651 {
          tunnel: w2603 -> [_ w2925 _ _]
          tunnel: w2604 -> [_ _ w2926 _]
          tunnel: [u32[][] [] ("24-bit pixmap") w2925 w2926 w2927] -> w2601
          tunnel: w2605 -> [_ _ _ w2927]
          frame 0, Default {
          }
          frame 1 {
          }
          frame 2 {
          }
          frame 3 {
          }
        }
        n2106 = case shown="0, Default" w2748 {
          tunnel: w2611 -> [_ w2959 _]
          tunnel: w2610 -> [_ _ w2960]
          tunnel: [u32[][] [] ("24-bit pixmap") w2959 w2960] -> w2764
          frame 0, Default {
          }
          frame 1 {
          }
          frame 2 {
          }
        }
        n2107 = case shown="0, Default" w2758 {
          tunnel: w2611 -> [_ w2953 _]
          tunnel: w2610 -> [_ _ w2954]
          tunnel: [u32[][] [] ("24-bit pixmap") w2953 w2954] -> w2766
          frame 0, Default {
          }
          frame 1 {
          }
          frame 2 {
          }
        }
        n2108 = case shown="0, Default" w2718 {
          tunnel: w2609 -> [_ w2947 _]
          tunnel: w2608 -> [_ _ w2948]
          tunnel: [u32[][] [] ("24-bit pixmap") w2947 w2948] -> w2702
          frame 0, Default {
          }
          frame 1 {
          }
          frame 2 {
          }
        }
        n2109 = case shown="0, Default" w2708 {
          tunnel: w2609 -> [_ w2941 _]
          tunnel: w2608 -> [_ _ w2942]
          tunnel: [u32[][] [] ("24-bit pixmap") w2941 w2942] -> w2700
          frame 0, Default {
          }
          frame 1 {
          }
          frame 2 {
          }
        }
        n2110 = case shown="0, Default" w2670 {
          tunnel: w2607 -> [_ w2938 _]
          tunnel: w2606 -> [_ _ w2939]
          tunnel: [u32[][] [] ("24-bit pixmap") w2938 w2939] -> w2691
          frame 0, Default {
          }
          frame 1 {
          }
          frame 2 {
          }
        }
        n2111 = case shown="0, Default" w2681 {
          tunnel: w2607 -> [_ w2932 _]
          tunnel: w2606 -> [_ _ w2933]
          tunnel: [u32[][] [] ("24-bit pixmap") w2932 w2933] -> w2693
          frame 0, Default {
          }
          frame 1 {
          }
          frame 2 {
          }
        }
        n2112 = case shown="0, Default" w2742 {
          tunnel: w2611 -> [_ w2962 _]
          tunnel: w2610 -> [_ _ w2963]
          tunnel: [u32[][] [] ("24-bit pixmap") w2962 w2963] -> w2763
          frame 0, Default {
          }
          frame 1 {
          }
          frame 2 {
          }
        }
        n2113 = case shown="0, Default" w2753 {
          tunnel: w2611 -> [_ w2956 _]
          tunnel: w2610 -> [_ _ w2957]
          tunnel: [u32[][] [] ("24-bit pixmap") w2956 w2957] -> w2765
          frame 0, Default {
          }
          frame 1 {
          }
          frame 2 {
          }
        }
        n2114 = case shown="0, Default" w2724 {
          tunnel: w2609 -> [_ w2950 _]
          tunnel: w2608 -> [_ _ w2951]
          tunnel: [u32[][] [] ("24-bit pixmap") w2950 w2951] -> w2703
          frame 0, Default {
          }
          frame 1 {
          }
          frame 2 {
          }
        }
        n2115 = case shown="0, Default" w2713 {
          tunnel: w2609 -> [_ w2944 _]
          tunnel: w2608 -> [_ _ w2945]
          tunnel: [u32[][] [] ("24-bit pixmap") w2944 w2945] -> w2701
          frame 0, Default {
          }
          frame 1 {
          }
          frame 2 {
          }
        }
        n2116 = case shown="3" w2640 {
          tunnel: w2603 -> [_ w2917 _ _]
          tunnel: w2604 -> [_ _ w2918 _]
          tunnel: [u32[][] [] ("24-bit pixmap") w2917 w2918 w2919] -> w2629
          tunnel: w2605 -> [_ _ _ w2919]
          frame 0, Default {
          }
          frame 1 {
          }
          frame 2 {
          }
          frame 3 {
          }
        }
        n2117 = case shown="3" w2635 {
          tunnel: w2603 -> [_ w2913 _ _]
          tunnel: w2604 -> [_ _ w2914 _]
          tunnel: [u32[][] [] ("24-bit pixmap") w2913 w2914 w2915] -> w2628
          tunnel: w2605 -> [_ _ _ w2915]
          frame 0, Default {
          }
          frame 1 {
          }
          frame 2 {
          }
          frame 3 {
          }
        }
        n2118 = call-poly <vilib>:"Draw Unflattened Pixmap.vi"("data (RGB format)"=w2620) -> ("new picture"=w2905:picture)  [unwired: 8 in]
        n2119 = call-poly <vilib>:"Draw Unflattened Pixmap.vi"("picture"=w2905, "top left point(0, 0)"=cluster{"x":i16, "y":i16} {"x"=1104, "y"=31}, "data (RGB format)"=w2904) -> ("new picture"=w2894:picture)  [unwired: 6 in]
        n2120 = call-poly <vilib>:"Draw Unflattened Pixmap.vi"("picture"=w2894, "top left point(0, 0)"=cluster{"x":i16, "y":i16} {"x"=779, "y"=31}, "data (RGB format)"=w2895) -> ("new picture"=w2887:picture)  [unwired: 6 in]
        n2121 = call-poly <vilib>:"Draw Unflattened Pixmap.vi"("picture"=w2887, "top left point(0, 0)"=cluster{"x":i16, "y":i16} {"x"=453, "y"=31}, "data (RGB format)"=w2879) -> ("new picture"=w2876:picture)  [unwired: 6 in]
        n2122 = call-poly <vilib>:"Draw Unflattened Pixmap.vi"("picture"=w2876, "top left point(0, 0)"=cluster{"x":i16, "y":i16} {"x"=127, "y"=31}, "data (RGB format)"=w2877) -> ("new picture"=w2849:picture)  [unwired: 6 in]
        n2123 = call-poly <vilib>:"Draw Unflattened Pixmap.vi"("picture"=w2849, "top left point(0, 0)"=cluster{"x":i16, "y":i16} {"x"=1076, "y"=146}, "data (RGB format)"=w2848) -> ("new picture"=w2846:picture)  [unwired: 6 in]
        n2124 = call-poly <vilib>:"Draw Unflattened Pixmap.vi"("picture"=w2846, "top left point(0, 0)"=cluster{"x":i16, "y":i16} {"x"=750, "y"=146}, "data (RGB format)"=w2847) -> ("new picture"=w2845:picture)  [unwired: 6 in]
        n2125 = call-poly <vilib>:"Draw Unflattened Pixmap.vi"("picture"=w2845, "top left point(0, 0)"=cluster{"x":i16, "y":i16} {"x"=424, "y"=146}, "data (RGB format)"=w2844) -> ("new picture"=w2842:picture)  [unwired: 6 in]
        n2126 = call-poly <vilib>:"Draw Unflattened Pixmap.vi"("picture"=w2842, "top left point(0, 0)"=cluster{"x":i16, "y":i16} {"x"=100, "y"=146}, "data (RGB format)"=w2843) -> ("new picture"=w2804:picture)  [unwired: 6 in]
        n2127 = call-poly <vilib>:"Draw Unflattened Pixmap.vi"("picture"=w2804, "top left point(0, 0)"=cluster{"x":i16, "y":i16} {"x"=1163, "y"=215}, "data (RGB format)"=w2831) -> ("new picture"=w2833:picture)  [unwired: 6 in]
        n2128 = call-poly <vilib>:"Draw Unflattened Pixmap.vi"("picture"=w2833, "top left point(0, 0)"=cluster{"x":i16, "y":i16} {"x"=838, "y"=216}, "data (RGB format)"=w2832) -> ("new picture"=w2834:picture)  [unwired: 6 in]
        n2129 = call-poly <vilib>:"Draw Unflattened Pixmap.vi"("picture"=w2834, "top left point(0, 0)"=cluster{"x":i16, "y":i16} {"x"=512, "y"=217}, "data (RGB format)"=w2835) -> ("new picture"=w2837:picture)  [unwired: 6 in]
        n2130 = call-poly <vilib>:"Draw Unflattened Pixmap.vi"("picture"=w2837, "top left point(0, 0)"=cluster{"x":i16, "y":i16} {"x"=186, "y"=216}, "data (RGB format)"=w2836) -> ("new picture"=w2660:picture)  [unwired: 6 in]
        n2131 = call-poly <vilib>:"Draw Unflattened Pixmap.vi"("picture"=w2660, "top left point(0, 0)"=cluster{"x":i16, "y":i16} {"x"=1180, "y"=150}, "data (RGB format)"=w2777) -> ("new picture"=w2775:picture)  [unwired: 6 in]
        n2132 = call-poly <vilib>:"Draw Unflattened Pixmap.vi"("picture"=w2775, "top left point(0, 0)"=cluster{"x":i16, "y":i16} {"x"=856, "y"=150}, "data (RGB format)"=w2776) -> ("new picture"=w2774:picture)  [unwired: 6 in]
        n2133 = call-poly <vilib>:"Draw Unflattened Pixmap.vi"("picture"=w2774, "top left point(0, 0)"=cluster{"x":i16, "y":i16} {"x"=530, "y"=150}, "data (RGB format)"=w2773) -> ("new picture"=w2771:picture)  [unwired: 6 in]